vi "UHR-Fleezers Control (host) - Avogadro v3.vi"() -> ()   [LabVIEW 2014] (continued)
        n2336 = Unbundle By Name(w3621) -> ("kappa_x (pN/nm)"=w3623:dbl, "kappa_y (pN/nm)"=w3622:dbl)
        n2337 = Unbundle By Name(w3629) -> ("Set 1"=w3632:dbl, "Set 2"=w3631:dbl)
        n2338 = case shown="True" "Scale intensities" {
          tunnel: w3632 -> [w3646 w3659]
          tunnel: w3631 -> [w3645 w3652]
          tunnel: "Scaling factor" -> [w3642 w3647]
          tunnel: [w3644 w3658] -> w3627
          tunnel: [w3643 w3657] -> w3626
          tunnel: w3625 -> [w3641 w3653]
          tunnel: w3624 -> [w3640 w3654]
          tunnel: w3623 -> [w3639 w3655]
          tunnel: w3622 -> [w3638 w3656]
          tunnel: [w3637 w3651] -> w3620
          tunnel: [w3636 w3650] -> w3619
          tunnel: [w3635 w3649] -> w3618
          tunnel: [w3634 w3648] -> w3617
          frame False {
            n2339 = Divide(x=w3646, y=w3642) -> (x/y=w3644:dbl)
            n2340 = Divide(x=w3638, y=w3642) -> (x/y=w3634:dbl)
            n2341 = Divide(x=w3645, y=w3642) -> (x/y=w3643:dbl)
            n2342 = Divide(x=w3641, y=w3642) -> (x/y=w3637:dbl)
            n2343 = Divide(x=w3640, y=w3642) -> (x/y=w3636:dbl)
            n2344 = Divide(x=w3639, y=w3642) -> (x/y=w3635:dbl)
          }
          frame True {
            n2345 = Multiply(x=w3659, y=w3647) -> (x*y=w3658:dbl)
            n2346 = Multiply(x=w3652, y=w3647) -> (x*y=w3657:dbl)
            n2347 = Multiply(x=w3656, y=w3647) -> (x*y=w3648:dbl)
            n2348 = Multiply(x=w3653, y=w3647) -> (x*y=w3651:dbl)
            n2349 = Multiply(x=w3654, y=w3647) -> (x*y=w3650:dbl)
            n2350 = Multiply(x=w3655, y=w3647) -> (x*y=w3649:dbl)
          }
        }
        n2351 = Bundle By Name(cluster=w3614, "kappa_x (pN/nm)"=w3620, "kappa_y (pN/nm)"=w3619) -> (w3616:T12)
        n2352 = Bundle By Name(cluster=w3621, "kappa_x (pN/nm)"=w3618, "kappa_y (pN/nm)"=w3617) -> (w3615:T12)
        n2353 = Bundle By Name(cluster=w3629, "Set 1"=w3627, "Set 2"=w3626) -> (w3628:cluster{"Set 1":dbl, "Set 2":dbl})
        n2354 = property on="T1 calibration" class="Clust (strict)"("Val(Sgnl)"=w3616) -> ()  [unwired: 2 in, 2 out]
        n2355 = property on="T2 calibration" class="Clust (strict)"("Val(Sgnl)"=w3615) -> ()  [unwired: 2 in, 2 out]
        n2356 = property on="Setpoints (V)" class="Clust (strict)"("Val(Sgnl)"=w3628) -> ()  [unwired: 2 in, 2 out]
      }
      event "Piezo X at\n Scan position (V)": Value Change {
        n2357 = event-data() -> ()  [unwired: 7 out]
        n2358 = local read "AOM position for scan (MHz)"() -> (w3668:dbl)
        n2359 = local read "Piezo Trap X cal (nm/V)"() -> (w3662:dbl)
        n2360 = local read "AOM X Cal (nm/MHz)"() -> (w3665:dbl)
        n2361 = Subtract(x=w3668, y=60.0) -> (x-y=w3666:dbl)
        n2362 = Multiply(x=w3666, y=w3665) -> (x*y=w3663:dbl)
        n2363 = Multiply(x="Piezo X at\n Scan position (V)", y=w3662) -> (x*y=w3664:dbl)
        n2364 = Subtract(x=w3664, y=w3663) -> (x-y=w3661:dbl)
        n2365 = Divide(x=w3661, y=w3662) -> (x/y=→"Piezo trap x\noffset (V)":dbl)
      }
      event "Shift offset": Value Change {
        # "This events shifts the offset values by the currently measured values. For a quick way of correcting for changes in offsets"
        n2366 = event-data() -> ()  [unwired: 7 out]
        n2367 = local read "Multi-MCL offset array"() -> (w3691:T31)
        n2368 = local read "Offset file step size"() -> (w3679:dbl)
        n2369 = local read "MCL offset scanning range (V)"() -> (w3680:T4)
        n2370 = local write "Shift offset"(FALSE) -> ()
        n2371 = local read "Trap position array"() -> (w3692:dbl[])
        n2372 = Build Array(1, 0, 4, 3, 11, 10) -> (w3683:i32[])
        n2373 = local read "Values"() -> (w3684:dbl[])
        n2374 = for {
          tunnel: w3684 -> [w3696]
          tunnel: w3683 -> [w3695] mode=indexing
          tunnel: [w3694] -> w3682 mode=indexing
          n2375 = Index Array(array=w3696, index=w3695) -> (element=w3694:dbl)
        }
        n2376 = call "select offset array.vi"("MCL offset scanning range (V)"=w3680, "Offset File step size"=w3679, "Multi-MCL offset array"=w3691, "Trap position array"=w3692) -> ("Out offsets"=w3681:dbl[])  [unwired: 1 out]
        n2377 = Subtract(x=w3682, y=w3681) -> (x-y=w3671:dbl[])
        n2378 = local read "Raw offsets"() -> (w3678:dbl[])
        n2379 = Negate(x=w3671) -> (-x=w3670:dbl[])
        n2380 = call "generate multiple MCL offset.vi"("Offset array"=w3678, "offset file step size"=w3679, "MCL offset scanning range (V)"=w3680, "Corrections"=w3670) -> ("B_X mean out"=w3672:dbl[], "A_X mean out"=w3673:dbl[], "Output array"=w3677:T31)
        n2381 = local write "Multi-MCL offset array"(w3677) -> ()
        n2382 = local read "B factor"() -> (w3674:dbl)
        n2383 = Multiply(x=w3672, y=w3674) -> (x*y=w3676:dbl[])
        n2384 = Subtract(x=w3673, y=w3676) -> (x-y=w3675:dbl[])
        n2385 = property on="Setpoint offset\ncorrection values" class="Arr (strict)"("Val(Sgnl)"=w3675) -> ()  [unwired: 2 in, 2 out]
      }
      event "Symmetric raster\nand force FB": Value Change {
        n2386 = event-data() -> ()  [unwired: 7 out]
        n2387 = local read "Symmetric raster\nand force FB"() -> (w3697:bool)
        n2388 = xnode "Read/Write Control"("FPGA VI Reference In"=w3698, "Symmetric force feedback and raster scan"=w3697) -> ()  [unwired: 1 in, 2 out]
      }
      event "EMCCD Gate", "EMCCD Gate ON Count", "EMCCD Gate OFF Count", "Invert EMCCD Gate": Value Change {
        n2389 = event-data() -> ()  [unwired: 7 out]
        n2390 = xnode "Read/Write Control"("FPGA VI Reference In"=w3703, "EMCCD Gate ON count"="EMCCD Gate ON Count", "EMCCD Gate OFF count"="EMCCD Gate OFF Count", "Invert EMCCD Gate"="Invert EMCCD Gate", "EMCCD Gate Operating Mode"="EMCCD Gate") -> ()  [unwired: 1 in, 2 out]
      }
      event "+ phase (EMCCD Gate)", "- phase (EMCCD Gate)": Value Change {
        n2391 = event-data() -> ()  [unwired: 7 out]
        n2392 = Or(x="- phase (EMCCD Gate)", y="+ phase (EMCCD Gate)") -> (x .or. y?=w3708:bool)
        n2393 = Negate(x="Phase Adj. (EMCCD Gate)") -> (-x=w3714:i16)
        n2394 = Select(t=w3714, s="+ phase (EMCCD Gate)", f="Phase Adj. (EMCCD Gate)") -> (s? t:f=w3709:i16)
        n2395 = flat-sequence {
          tunnel: w3710 -> [w3718]
          tunnel: w3709 -> [w3717]
          tunnel: [w3716] -> w3707
          tunnel: [w3715] -> w3705
          tunnel: w3708 -> [w3715]
          tunnel: w3707 -> [w3721]
          tunnel: [w3721] -> w3706
          tunnel: w3705 -> [w3720]
          tunnel: [w3720] -> w3704
          tunnel: w3706 -> [w3723]
          tunnel: w3704 -> [w3722]
          frame #0 {
            n2396 = xnode "Read/Write Control"("FPGA VI Reference In"=w3718, "Phase Count Adjustment EMCCD Gate"=w3717) -> ("FPGA VI Reference Out"=w3716:T41)  [unwired: 1 in, 1 out]
          }
          frame #1 {
            n2397 = Wait (ms)(milliseconds to wait=100) -> ()  [unwired: 1 out]
          }
          frame #2 {
            n2398 = xnode "Read/Write Control"("FPGA VI Reference In"=w3723, "+ phase (EMCCD Gate)"=w3722) -> ()  [unwired: 1 in, 2 out]
          }
        }
      }
    }
    "error out 2" <- w1836
    n2399 = node-c288() -> ()  [unwired: 2 out]
  }
  n2400 = node-c288() -> (w64:T43)  [unwired: 4 out]
  n2401 = timed-loop "Mouse control: trap position (AOM deflection), set confocal spot from image" {
    tunnel: [w3724] -> w69
    timing: w64 -> [_]
    timing-out: [_] -> w63
    tunnel: w26 -> [w3725]
    stop <- w3724 stop-if-true
    n2402 = node-c288() -> ()  [unwired: 2 out]
    n2403 = event shown="[0] \"Pane\": Mouse Down" {
      selector: _ -> [_ _ _ _]
      dyn-events: _ -> [_ _ _ _]
      timeout: _ -> [_ _ _ _]
      tunnel: w3725 -> [w3728 _ _ _]
      tunnel: [_ _ TRUE _] -> w3724
      event Mouse Down {
        n2404 = event-data() -> ("Time"=w3730:u32, "Coords"=w3729:T16, "Button"=w3731:u16)  [unwired: 6 out]
        n2405 = case shown="1" w3731 {
          tunnel: w3730 -> [_ _ w3861]
          tunnel: w3729 -> [_ w3768 w3859]
          tunnel: w3728 -> [_ _ w3855]
          frame 0, Default {
          }
          frame 1 {
            n2406 = property on="APD 2" class="ImageControl"() -> ("Displayed Image Position"=w3738:cluster{"Left":i32, "Top":i32})  [unwired: 2 in, 2 out]
            n2407 = property on="APD 1" class="ImageControl"() -> ("Displayed Image Position"=w3767:cluster{"Left":i32, "Top":i32})  [unwired: 2 in, 2 out]
            n2408 = property on="Detection Laser X" class="ImageControl"() -> ("Displayed Image Position"=w3764:cluster{"Left":i32, "Top":i32})  [unwired: 2 in, 2 out]
            n2409 = property on="Detection Laser Y" class="ImageControl"() -> ("Displayed Image Position"=w3763:cluster{"Left":i32, "Top":i32})  [unwired: 2 in, 2 out]
            n2410 = property on="APD 2" class="ImageControl"() -> ("Displayed Image Size"=w3737:cluster{"Width":u32, "Height":u32})  [unwired: 2 in, 2 out]
            n2411 = property on="APD 1" class="ImageControl"() -> ("Displayed Image Size"=w3765:cluster{"Width":u32, "Height":u32})  [unwired: 2 in, 2 out]
            n2412 = property on="Detection Laser X" class="ImageControl"() -> ("Displayed Image Size"=w3766:cluster{"Width":u32, "Height":u32})  [unwired: 2 in, 2 out]
            n2413 = property on="Detection Laser Y" class="ImageControl"() -> ("Displayed Image Size"=w3762:cluster{"Width":u32, "Height":u32})  [unwired: 2 in, 2 out]
            n2414 = Unbundle By Name(w3737) -> ("Width"=w3734:u32, "Height"=w3733:u32)
            n2415 = Unbundle By Name(w3738) -> ("Left"=w3736:i32, "Top"=w3735:i32)
            n2416 = Unbundle By Name(w3765) -> ("Width"=w3759:u32, "Height"=w3758:u32)
            n2417 = Unbundle By Name(w3766) -> ("Width"=w3755:u32, "Height"=w3754:u32)
            n2418 = Unbundle By Name(w3762) -> ("Width"=w3751:u32, "Height"=w3750:u32)
            n2419 = Unbundle By Name(w3767) -> ("Left"=w3761:i32, "Top"=w3760:i32)
            n2420 = Unbundle By Name(w3764) -> ("Left"=w3757:i32, "Top"=w3756:i32)
            n2421 = Unbundle By Name(w3763) -> ("Left"=w3753:i32, "Top"=w3752:i32)
            n2422 = Bundle("Left"=w3736, "Top"=w3735, "Width"=w3734, "Height"=w3733) -> (w3732:T59)  [unwired: 1 in]
            n2423 = Bundle("Left"=w3761, "Top"=w3760, "Width"=w3759, "Height"=w3758) -> (w3749:T59)  [unwired: 1 in]
            n2424 = Bundle("Left"=w3757, "Top"=w3756, "Width"=w3755, "Height"=w3754) -> (w3748:T59)  [unwired: 1 in]
            n2425 = Bundle("Left"=w3753, "Top"=w3752, "Width"=w3751, "Height"=w3750) -> (w3747:T59)  [unwired: 1 in]
            n2426 = Build Cluster Array(w3732, w3749, w3748, w3747) -> (w3746:T60)
            n2427 = for {
              tunnel: w3768 -> [w3779]
              tunnel: w3746 -> [w3780] mode=indexing
              shift-right: [w3777] -> w3744
              shift-left: TRUE -> [w3778]
              shift-right: [w3776] -> w3742
              shift-left: _ -> [w3772]
              shift-right: [w3775] -> w3741
              shift-left: _ -> [w3771]
              shift-right: [w3774] -> w3740
              shift-left: _ -> [w3770]
              shift-right: [w3773] -> w3739
              shift-left: _ -> [w3769]
              n2428 = case shown="True" w3778 {
                selector: w3778 -> [w3785 _]
                tunnel: w3780 -> [_ w3794]
                tunnel: w3779 -> [_ w3792]
                tunnel: [w3785 w3790] -> w3777
                tunnel: [w3784 w3789] -> w3776
                tunnel: [w3783 w3788] -> w3775
                tunnel: [w3782 w3787] -> w3774
                tunnel: [w3781 w3786] -> w3773
                tunnel: w3772 -> [w3784 _]
                tunnel: w3771 -> [w3783 _]
                tunnel: w3770 -> [w3782 _]
                tunnel: w3769 -> [w3781 _]
                frame False {
                }
                frame True {
                  n2429 = Unbundle(w3794) -> (w3793:T59)
                  n2430 = call "isclickinwindow.vi"("Image Param"=w3793, "Point32"=w3792) -> ("4 Y"=w3786:i32, "3 Height"=w3787:i32, "2 X"=w3788:i32, "1 Width"=w3789:i32, "In image?"=w3791:bool)  [unwired: 1 in]
                  n2431 = Not(x=w3791) -> (.not. x?=w3790:bool)
                }
              }
            }
            n2432 = Not(x=w3744) -> (.not. x?=w3743:bool)
            n2433 = case shown="True" w3743 {
              tunnel: w3741 -> [_ w3820]
              tunnel: w3739 -> [_ w3819]
              tunnel: w3742 -> [_ w3818]
              tunnel: w3740 -> [_ w3817]
              frame False {
              }
              frame True {
                w3807 = FALSE ("Get Point")
                n2434 = local read "Scan lines (y)"() -> (w3800:u64)
                n2435 = local read "Initial Y"() -> (w3798:dbl)
                n2436 = local read "Actual MCL Inc (V)"() -> (w3801:dbl)
                n2437 = local read "Scan steps (MCL)"() -> (w3804:u64)
                n2438 = local read "Actual MCL Inc (V)"() -> (w3816:dbl)
                n2439 = local read "Scan lines (y)"() -> (w3821:u64)
                n2440 = Divide "Y Pix/step"(x=w3817, y=w3821) -> (x/y=w3827:dbl)
                n2441 = Multiply(x=w3801, y=w3800) -> (x*y=w3799:dbl)
                n2442 = Divide "X pix/step"(x=w3818, y=w3804) -> (x/y=w3825:dbl)
                n2443 = Add(x=w3799, y=w3798) -> (x+y=w3797:dbl)
                n2444 = Divide "Y V/pix"(x=w3816, y=w3827) -> (x/y=w3826:dbl)
                n2445 = Divide "Y half step offset"(x=w3816, y=2.0) -> (x/y=w3803:dbl)
                n2446 = Divide "X half step offset"(x=w3816, y=2.0) -> (x/y=w3823:dbl)
                n2447 = Divide "X V/pix"(x=w3816, y=w3825) -> (x/y=w3824:dbl)
                n2448 = Multiply(x=w3819, y=w3826) -> (x*y=w3796:dbl)
                n2449 = Negate(x=w3796) -> (-x=w3795:dbl)
                n2450 = Negate(x=w3803) -> (-x=w3802:dbl)
                n2451 = Multiply(x=w3816, y=w3804) -> (x*y=w3829:dbl)
                n2452 = Multiply(x=w3824, y=w3820) -> (x*y=w3831:dbl)
                n2453 = Negate(x=w3823) -> (-x=w3822:dbl)
                n2454 = Compound Arithmetic op=ADD(w3802, w3795, w3797) -> (w3808:dbl)
                "Pointer Y (V)" <- w3808
                n2455 = local read "Initial X"() -> (w3832:dbl)
                n2456 = Negate(x=w3831) -> (-x=w3830:dbl)
                n2457 = Compound Arithmetic op=ADD(w3822, w3829, w3832, w3830) -> (w3809:dbl)
                "Pointer X (V)" <- w3809
                n2458 = case shown="True" "Set High F Confocal Spot (X-Y)" {
                  tunnel: w3809 -> [_ w3853]
                  tunnel: w3808 -> [_ w3854]
                  frame False {
                  }
                  frame True {
                    "Confocal Y 2 (V)" <- w3854
                    "Confocal X 2 (V)" <- w3853
                  }
                }
                n2459 = local read "Scan trap 3 or Fl?"() -> (w3806:bool)
                n2460 = Or(x="Set X Only", y="Set Confocal Spot (X-Y)") -> (x .or. y?=w3812:bool)
                n2461 = Or(x="Set Confocal Spot (X-Y)", y="Set Y Only") -> (x .or. y?=w3811:bool)
                n2462 = case shown="False" w3806 {
                  tunnel: w3812 -> [w3836 w3842]
                  tunnel: w3811 -> [w3835 w3841]
                  tunnel: w3809 -> [w3834 w3839]
                  tunnel: w3808 -> [w3833 w3840]
                  frame False {
                    n2463 = case shown="True" w3835 {
                      tunnel: w3833 -> [_ w3838]
                      frame False {
                      }
                      frame True {
                        n2464 = property on="AO1" class="Slide (strict)"("Val(Sgnl)"=w3838) -> ()  [unwired: 2 in, 2 out]
                        "Confocal Y 1 (V)" <- w3838
                      }
                    }
                    n2465 = case shown="True" w3836 {
                      tunnel: w3834 -> [_ w3837]
                      frame False {
                      }
                      frame True {
                        n2466 = property on="AO2" class="Slide (strict)"("Val(Sgnl)"=w3837) -> ()  [unwired: 2 in, 2 out]
                        "Confocal X 1 (V)" <- w3837
                      }
                    }
                  }
                  frame True {
                    n2467 = case shown="True" w3841 {
                      tunnel: w3840 -> [_ w3843]
                      frame False {
                      }
                      frame True {
                        n2468 = property on="Piezo trap y\noffset (V)" class="DigNum (strict)"("Val(Sgnl)"=w3843) -> ()  [unwired: 2 in, 2 out]
                      }
                    }
                    n2469 = case shown="True" w3842 {
                      tunnel: w3839 -> [_ w3848]
                      frame False {
                      }
                      frame True {
                        n2470 = local read "AOM X Cal (nm/MHz)"() -> (w3849:dbl)
                        n2471 = local read "Trap Delta (MHz)"() -> (w3851:dbl)
                        n2472 = Subtract(x=30.0, y=w3851) -> (x-y=w3850:dbl)
                        n2473 = Multiply(x=w3850, y=w3849) -> (x*y=w3846:dbl)
                        n2474 = local read "Piezo Trap X cal (nm/V)"() -> (w3845:dbl)
                        n2475 = Divide(x=w3846, y=w3845) -> (x/y=w3844:dbl)
                        n2476 = Subtract(x=w3848, y=w3844) -> (x-y=w3847:dbl)
                        n2477 = property on="Piezo trap x\noffset (V)" class="DigNum (strict)"("Val(Sgnl)"=w3847) -> ()  [unwired: 2 in, 2 out]
                      }
                    }
                  }
                }
                n2478 = local write "Set High F Confocal Spot (X-Y)"(w3807) -> ()
                n2479 = local write "Set Confocal Spot (X-Y)"(w3807) -> ()
                n2480 = local write "Set X Only"(w3807) -> ()
                n2481 = local write "Set Y Only"(w3807) -> ()
              }
            }
          }
          frame 3 {
            n2482 = local read "BD 2 Frequency 1 (MHz)"() -> (w3856:dbl)
            n2483 = local read "BD 1 Frequency 1 (MHz)"() -> (w3857:dbl)
            n2484 = local write "Manipulating Trap"(TRUE ("Manipulating Trap")) -> ()
            n2485 = local write "Coords"(T16 {"Horizontal"=0, "Vertical"=0} ("Coords")) -> ()
            n2486 = while {
              tunnel: w3861 -> [w3866]
              tunnel: w3859 -> [w3865]
              tunnel: w3857 -> [w3864]
              tunnel: w3856 -> [w3863]
              tunnel: w3855 -> [w3862]
              stop <- w3867 stop-if-true
              n2487 = event shown="[0] \"Pane\": Mouse Move" {
                selector: _ -> [_ _]
                dyn-events: _ -> [_ _]
                timeout: _ -> [_ _]
                tunnel: ["Force Manip Abort" w3931] -> w3867
                tunnel: w3866 -> [w3874 _]
                tunnel: w3865 -> [w3872 _]
                tunnel: w3864 -> [w3871 _]
                tunnel: w3863 -> [w3870 _]
                tunnel: w3862 -> [w3868 _]
                event Mouse Move {
                  n2488 = event-data() -> ("Time"=w3875:u32, "Coords"=w3876:T16)  [unwired: 3 out]
                  n2489 = Less?(x=w3875, y=w3874) -> (x < y?=w3873:bool)
                  n2490 = case "Makes sure old motion events prior to mouse click aren't used" shown="False" w3873 {
                    tunnel: w3876 -> [w3918 _]
                    tunnel: w3872 -> [w3919 _]
                    tunnel: w3871 -> [w3893 _]
                    tunnel: w3870 -> [w3892 _]
                    tunnel: w3868 -> [w3877 _]
                    frame False {
                      n2491 = Subtract(x=w3918, y=w3919) -> (x-y=w3917:T16)
                      "Coords" <- w3917
                      n2492 = local read "Y RF Frequency Limits (MHz)"() -> (w3878:T27)
                      n2493 = To Double Precision Float(number=w3917) -> (double precision float=w3916:cluster{"Horizontal":dbl, "Vertical":dbl})
                      n2494 = Multiply(x=cluster{"Horizontal":dbl, "Vertical":dbl} {"Horizontal"=-1.0, "Vertical"=1.0}, y="Manipulation Scaling") -> (x*y=w3912:cluster{"Horizontal":dbl, "Vertical":dbl})
                      n2495 = local read "X RF Frequency Limits (MHz)"() -> (w3879:T27)
                      n2496 = Multiply(x=w3916, y=w3912) -> (x*y=w3914:cluster{"Horizontal":dbl, "Vertical":dbl})
                      n2497 = Unbundle By Name(w3914) -> ("Horizontal"=w3909:dbl, "Vertical"=w3913:dbl)
                      n2498 = Unbundle By Name(w3878) -> ("Maximum"=w3881:dbl, "Minimum"=w3880:dbl)
                      n2499 = Boolean To (0,1)(Boolean="Manip. X?") -> (0, 1=w3907:i16)
                      n2500 = Boolean To (0,1)(Boolean="Manip. Y?") -> (0, 1=w3904:i16)
                      n2501 = local read "BD 1 Frequency 2 (MHz)"() -> (w3895:dbl)
                      n2502 = Multiply(x=w3913, y=w3904) -> (x*y=w3906:dbl)
                      n2503 = Multiply(x=w3907, y=w3909) -> (x*y=w3910:dbl)
                      n2504 = local read "BD 2 Frequency 2 (MHz)"() -> (w3894:dbl)
                      n2505 = Unbundle By Name(w3879) -> ("Maximum"=w3883:dbl, "Minimum"=w3882:dbl)
                      n2506 = Add(x=w3892, y=w3906) -> (x+y=w3885:dbl)
                      n2507 = Add(x=w3893, y=w3910) -> (x+y=w3887:dbl)
                      n2508 = In Range and Coerce(upper limit=w3883, x=w3887, lower limit=w3882) -> (coerced(x)=w3886:dbl)  [unwired: 1 out]
                      n2509 = In Range and Coerce(upper limit=w3881, x=w3885, lower limit=w3880) -> (coerced(x)=w3884:dbl)  [unwired: 1 out]
                      n2510 = Subtract(x=w3886, y=w3895) -> (x-y=w3903:dbl)
                      n2511 = Subtract(x=w3884, y=w3894) -> (x-y=w3902:dbl)
                      n2512 = Square(x=w3903) -> (x^2=w3901:dbl)
                      n2513 = Square(x=w3902) -> (x^2=w3900:dbl)
                      n2514 = Add(x=w3901, y=w3900) -> (x+y=w3899:dbl)
                      n2515 = Square Root(x=w3899) -> (sqrt(x)=w3896:dbl)
                      n2516 = In Range and Coerce(upper limit="Limit Max (MHz)", x=w3896, lower limit="Limit Min (MHz)") -> (In Range?=w3889:bool)  [unwired: 1 out]
                      n2517 = Not(x="Limits Enable") -> (.not. x?=w3888:bool)
                      n2518 = Or(x=w3889, y=w3888) -> (x .or. y?=w3890:bool)
                      n2519 = case shown="True" w3890 {
                        tunnel: w3896 -> [_ w3921]
                        tunnel: w3886 -> [_ w3928]
                        tunnel: w3895 -> [_ w3927]
                        tunnel: w3884 -> [_ w3926]
                        tunnel: w3894 -> [_ w3925]
                        tunnel: w3879 -> [_ w3923]
                        tunnel: w3878 -> [_ w3922]
                        tunnel: w3877 -> [_ w3920]
                        frame False {
                        }
                        frame True {
                          n2520 = local read "BD 1 Frequency 3 (MHz)"() -> (w3929:dbl)
                          n2521 = local read "BD 2 Frequency 3 (MHz)"() -> (w3924:dbl)
                          n2522 = local write "Trap Delta (MHz)"(w3921) -> ()
                          n2523 = call "set RF board frequency - interlace.vi"("Board 2 Frequency Limits"=w3922, "Board 1 Frequency Limits"=w3923, "FPGA VI Reference In"=w3920, "Board 2 Frequency 3 (MHz)"=w3924, "Board 1 Frequency 3 (MHz)"=w3929, "Board 2 Frequency 2 (MHz)"=w3925, "Board 2 Frequency 1 (MHz)"=w3926, "Board 1 Frequency 2 (MHz)"=w3927, "Board 1 Frequency 1  (MHz)"=w3928) -> ()  [unwired: 1 in, 2 out]
                          n2524 = local write "BD 2 Frequency 1 (MHz)"(w3926) -> ()
                          n2525 = local write "BD 1 Frequency 1 (MHz)"(w3928) -> ()
                        }
                      }
                    }
                    frame True {
                    }
                  }
                }
                event Mouse Up {
                  n2526 = event-data() -> ("Button"=w3930:u16)  [unwired: 8 out]
                  n2527 = case shown="3" w3930 {
                    tunnel: [FALSE TRUE] -> w3931
                    frame 0, Default {
                    }
                    frame 3 {
                      n2528 = local read "Trap Delta (MHz)"() -> (w3933:dbl)
                      n2529 = property on="Initial delta (MHz)" class="DigNum (strict)"("Val(Sgnl)"=w3933) -> ()  [unwired: 2 in, 2 out]
                      n2530 = local write "Manipulating Trap"(FALSE ("Manipulating Trap")) -> ()
                    }
                  }
                }
              }
            }
          }
        }
      }
      event Timeout {
        n2531 = event-data() -> ()  [unwired: 4 out]
      }
      event "Stop All": Mouse Down {
        n2532 = event-data() -> ()  [unwired: 9 out]
      }
      event Mouse Move {
        n2533 = event-data() -> ()  [unwired: 6 out]
      }
    }
    n2534 = node-c288() -> ()  [unwired: 2 out]
  }
  n2535 = node-c288(i64 1 ("Period"), 1 ("Processor")) -> (w68:T43)  [unwired: 2 in, 2 out]
  n2536 = node-c288(3 ("Processor")) -> (w60:T43)  [unwired: 3 out]
  n2537 = timed-loop "Oscillate Trap/AOM (fishing, conjugate plane alignment)" {
    tunnel: [w3939] -> w65
    timing: w60 -> [_]
    timing-out: [_] -> w59
    tunnel: w26 -> [w3938]
    tunnel: w3 -> [w3937]
    stop <- w3939 stop-if-true
    n2538 = node-c288() -> ()  [unwired: 2 out]
    n2539 = event shown="[2] \"Start assembly line\": Value Change" {
      selector: _ -> [_ _ _ _]
      dyn-events: _ -> [_ _ _ _]
      timeout: _ -> [_ _ _ _]
      tunnel: [FALSE ("Stop All") _ _ w4612] -> w3939
      tunnel: w3938 -> [w3942 _ _ _]
      tunnel: w3937 -> [_ _ w4547 _]
      event "Oscillate Set 1", "Fish for Tether": Value Change {
        n2540 = event-data() -> ()  [unwired: 6 out]
        n2541 = local read "Oscillate Set 1"() -> (w3946:bool)
        n2542 = Or(x=w3946, y="Fish for Tether") -> (x .or. y?=w3944:bool)
        n2543 = case shown="True" w3944 {
          tunnel: "Fish for Tether" -> [_ w3949]
          tunnel: w3942 -> [_ w3947]
          frame False {
          }
          frame True {
            n2544 = case shown="True" w3949 {
              selector: w3949 -> [w3952 w3958]
              tunnel: [w3952 w3958] -> w3948
              frame False {
              }
              frame True {
                n2545 = local write "Scan axis 2"(TRUE) -> ()
                n2546 = local write "Tether"(FALSE ("Tether")) -> ()
                n2547 = local read "Flow ON during cal?"() -> (w3953:bool)
                n2548 = property on="Trap Delta (MHz)" class="DigNum (strict)"("Val(Sgnl)"="Furthest Delta (MHz)") -> ()  [unwired: 2 in, 2 out]
                n2549 = Or(x="Flow ON during \nfishing?", y=w3953) -> (x .or. y?=w3954:bool)
                n2550 = Wait (ms)(milliseconds to wait=u32 500) -> ()  [unwired: 1 out]
                n2551 = property on="Sample Channel\nFlow" class="Bool (strict)"("Val(Sgnl)"=w3954) -> ()  [unwired: 2 in, 2 out]
              }
            }
            n2552 = node-c288() -> (w3951:T43)  [unwired: 1 in, 3 out]
            n2553 = timed-loop "Oscillate AOD" {
              timing: w3951 -> [_]
              timing-out: [_] -> w3950
              tunnel: w3948 -> [w3962]
              tunnel: w3947 -> [w3961]
              i -> [w3970]
              stop <- w3968 stop-if-true
              n2554 = node-c288() -> (w3969:i64)  [unwired: 1 out]
              n2555 = flat-sequence {
                tunnel: w3970 -> [w3997]
                tunnel: w3969 -> [w3996]
                tunnel: w3962 -> [w3980]
                tunnel: [w3980] -> w3967
                tunnel: [w3979] -> w3966
                tunnel: [w3978] -> w3965
                tunnel: [w3975] -> w3963
                tunnel: w3961 -> [w3971]
                tunnel: w3967 -> [w4044]
                tunnel: w3966 -> [w4042]
                tunnel: w3965 -> [w4041]
                tunnel: [w4040] -> w3964
                tunnel: w3963 -> [w4039]
                tunnel: [w4116] -> w3968
                tunnel: w3964 -> [w4115]
                frame #0 {
                  # "w (rad/s)"
                  # "t (s)"
                  n2556 = Divide(x=w3996, y=i64 1000) -> (x/y=w3972:dbl)
                  n2557 = local read "BD 1 Frequency 2 (MHz)"() -> (w3974:dbl)
                  n2558 = Multiply(x="Osc. freq. (Hz)", y=6.283185307179586) -> (x*y=w3994:dbl)
                  n2559 = Multiply(x=w3972, y=w3997) -> (x*y=w3993:dbl)
                  n2560 = Multiply(x=w3994, y=w3993) -> (x*y=w3977:dbl)
                  n2561 = local read "BD 1 Frequency 1 (MHz)"() -> (w3982:dbl)
                  n2562 = case shown="True" w3980 {
                    tunnel: w3977 -> [w4003 w4022]
                    tunnel: w3982 -> [_ w4030]
                    tunnel: w3974 -> [_ w4031]
                    tunnel: [w4000 w4026] -> w3973
                    tunnel: [FALSE w4004] -> w3978
                    tunnel: [0.0 w4018] -> w3975
                    frame False {
                      n2563 = Sine(x=w4003) -> (sin(x)=w4001:dbl)
                      n2564 = Multiply(x=w4001, y="Osc. amp. (MHz)") -> (x*y=w4000:dbl)
                    }
                    frame True {
                      # "trap position goes from 0 to 1 (0 is when it is furthest away, 1 is when closest)\nso we want to test for tether only when farther away, or x < 1"
                      # "quit if taking too long"
                      # "oscillate the trap"
                      # "Test for tether"
                      n2565 = local read "Vec Mean of T1 T2"() -> (w4007:dbl[])
                      "Trigger Signal" <- w4007
                      n2566 = Cosine(x=w4022) -> (cos(x)=w4034:dbl)
                      n2567 = Subtract(x=w4031, y=w4030) -> (x-y=w4029:dbl)
                      n2568 = Decrement(x=w4034) -> (x-1=w4033:dbl)
                      n2569 = Subtract(x=w4029, y="Closest Delta (MHz)") -> (x-y=w4027:dbl)
                      n2570 = Divide(x=w4033, y=-2.0) -> (x/y=w4017:dbl)
                      n2571 = Greater?(x=w4007, y="Stop F (pN)") -> (0:w4024:bool[])
                      n2572 = Multiply(x=w4017, y=w4027) -> (x*y=w4026:dbl)
                      n2573 = Less?(x=w4017, y="Fish mask thresh") -> (x < y?=w4016:bool)
                      n2574 = Boolean To (0,1)(Boolean=w4016) -> (0, 1=w4014:i16)
                      n2575 = Multiply(x=w4014, y=w4007) -> (x*y=w4013:dbl[])
                      n2576 = Divide(x=w4022, y=6.283185307179586) -> (x/y=w4021:dbl)
                      n2577 = Round Toward +Infinity(x=w4021) -> (ceil(x): smallest int >= x=w4018:dbl)
                      "Attempts" <- w4018
                      n2578 = Greater?(x=w4013, y="Stop F (pN) (mask)") -> (0:w4011:bool[])
                      n2579 = Or Array Elements(Boolean array=w4024) -> (logical OR=w4009:bool)
                      n2580 = Or Array Elements(Boolean array=w4011) -> (logical OR=w4008:bool)
                      n2581 = Greater?(x=w4018, y="Attempt Limit") -> (0:w4020:bool)
                      n2582 = case shown="True" w4020 {
                        frame False {
                        }
                        frame True {
                          n2583 = local write "Fish for Tether"(FALSE ("Fish for Tether")) -> ()
                          n2584 = call <vilib>:"Beep.vi"() -> ()  [unwired: 3 in, 9 out]
                          n2585 = local read "Messages"() -> (w4036:string)
                          n2586 = call "Update messages.vi"("Message to add"="Tether fishing timeout." ("Messages"), "Old message string"=w4036) -> ("New message string"=→"Messages":string)
                        }
                      }
                      n2587 = Select(t=w4009, s="Normal (on) or masked test (off)", f=w4008) -> (s? t:f=w4006:bool)
                      n2588 = And(x="Stop Fishing When Tether", y=w4006) -> (x .and. y?=w4004:bool)
                    }
                  }
                  n2589 = local read "BD 2 Frequency 1 (MHz)"() -> (w3981:dbl)
                  n2590 = Select(t=w3982, s="Scan axis 2", f=w3981) -> (s? t:f=w3985:dbl)
                  n2591 = Add(x=w3973, y=w3985) -> (x+y=w3979:dbl)
                  n2592 = Select(t=w3979, s="Scan axis 2", f=w3982) -> (s? t:f=w3988:dbl)
                  n2593 = Select(t=w3981, s="Scan axis 2", f=w3979) -> (s? t:f=w3987:dbl)
                  n2594 = local read "BD 2 Frequency 2 (MHz)"() -> (w3990:dbl)
                  n2595 = local read "BD 2 Frequency 3 (MHz)"() -> (w3989:dbl)
                  n2596 = local read "Y RF Frequency Limits (MHz)"() -> (w3983:T27)
                  n2597 = local read "X RF Frequency Limits (MHz)"() -> (w3984:T27)
                  n2598 = local read "BD 1 Frequency 3 (MHz)"() -> (w3991:dbl)
                  n2599 = call "set RF board frequency - interlace.vi"("Board 2 Frequency Limits"=w3983, "Board 1 Frequency Limits"=w3984, "FPGA VI Reference In"=w3971, "Board 2 Frequency 3 (MHz)"=w3989, "Board 1 Frequency 3 (MHz)"=w3991, "Board 2 Frequency 2 (MHz)"=w3990, "Board 2 Frequency 1 (MHz)"=w3987, "Board 1 Frequency 2 (MHz)"=w3974, "Board 1 Frequency 1  (MHz)"=w3988) -> ()  [unwired: 1 in, 2 out]
                }
                frame #1 {
                  n2600 = And(x=w4044, y=w4041) -> (x .and. y?=w4043:bool)
                  n2601 = case "Only if were fishing and now formed tether" shown="True" w4043 {
                    tunnel: w4042 -> [w4046 w4061]
                    tunnel: [w4045 w4060] -> w4040
                    tunnel: w4039 -> [_ w4056]
                    frame False {
                      n2602 = local read "Fish for Tether"() -> (w4045:bool)
                      n2603 = case shown="False" w4045 {
                        tunnel: w4046 -> [w4047 _]
                        frame False {
                          n2604 = property on="BD 1 Frequency 1 (MHz)" class="DigNum (strict)"("Val(Sgnl)"=w4047) -> ()  [unwired: 2 in, 2 out]
                        }
                        frame True {
                        }
                      }
                    }
                    frame True {
                      w4060 = FALSE ("Fish for Tether")
                      n2605 = call <vilib>:"Beep.vi"() -> ()  [unwired: 3 in, 9 out]
                      n2606 = Number To Decimal String(number=w4056, width (-)=i16 1) -> (decimal integer string=w4054:string)
                      n2607 = Concatenate Strings("Formed tether in ", w4054, " attempt(s)." ("string")) -> (w4051:string)
                      n2608 = local read "Messages"() -> (w4058:string)
                      n2609 = local write "Fish for Tether"(w4060) -> ()
                      n2610 = call "Update messages.vi"("Message to add"=w4051, "Old message string"=w4058) -> ("New message string"=w4057:string)
                      n2611 = local write "Messages"(w4057) -> ()
                      n2612 = Get Date/Time In Seconds() -> (seconds since 1Jan1904=→"Time tether formed":timestamp)
                      n2613 = local read "Flow ON during cal?"() -> (w4048:bool)
                      n2614 = property on="Sample Channel\nFlow" class="Bool (strict)"("Val(Sgnl)"=w4048) -> (error out=w4049:errorcluster)  [unwired: 2 in, 1 out]
                      n2615 = case shown="\"2\", \"3\", \"4\", \"5\", \"6\"" "Then..." {
                        selector: "Then..." -> [_ w4064]
                        tunnel: w4061 -> [w4063 _]
                        tunnel: w4049 -> [_ _]
                        frame "1", Default {
                          n2616 = property on="BD 1 Frequency 1 (MHz)" class="DigNum (strict)"("Val(Sgnl)"=w4063) -> ()  [unwired: 2 in, 2 out]
                        }
                        frame "2", "3", "4", "5", "6" {
                          n2617 = flat-sequence {
                            tunnel: w4064 -> [w4066]
                            frame #0 {
                              n2618 = property on="Trap Delta (MHz)" class="DigNum (strict)"("Val(Sgnl)"="Move to Delta 1 (MHz)") -> ()  [unwired: 2 in, 2 out]
                            }
                            frame #1 {
                              n2619 = case shown="\"5\", \"6\"" w4066 {
                                selector: w4066 -> [w4069 w4079 _]
                                frame "3", "4" {
                                n2620 = flat-sequence {
                                tunnel: w4069 -> [w4070]
                                tunnel: [w4070] -> w4067
                                tunnel: [w4072] -> w4068
                                tunnel: w4067 -> [w4072]
                                tunnel: w4068 -> [w4076]
                                frame #0 {
                                n2621 = property on="Vortran Laser ON" class="Bool (strict)"("Val(Sgnl)"=TRUE ("Value (Signaling)")) -> ()  [unwired: 2 in, 2 out]
                                }
                                frame #1 {
                                n2622 = Multiply(x="Wait Before Save (s)", y=u32 1000 ("x")) -> (x*y=w4074:u32)
                                n2623 = Wait (ms)(milliseconds to wait=w4074) -> ()  [unwired: 1 out]
                                }
                                frame #2 {
                                n2624 = property on="Start Saving" class="Bool (strict)"("Value"=TRUE ("Start Saving")) -> ()  [unwired: 2 in, 2 out]
                                n2625 = case shown="\"4\"" w4076 {
                                frame Default {
                                }
                                frame "4" {
                                n2626 = property on="Fl. Triggered..." class="Bool (strict)"("Val(Sgnl)"=TRUE ("Value (Signaling)")) -> ()  [unwired: 2 in, 2 out]
                                }
                                }
                                }
                                }
                                }
                                frame "5", "6" {
                                n2627 = stacked-sequence {
                                tunnel: w4079 -> [_ _ _ _ _ _ w4091]
                                frame #0 {
                                n2628 = Replace Array Subset(array=u32[] [0] ("Index Values"), new element="Raster Set Upon Tether", index=0) -> (w4080:u32[])
                                n2629 = property on="Saved AOD Raster Scan Parameter Sets" class="Arr (strict)"("Index Values"=w4080) -> ()  [unwired: 2 in, 2 out]
                                }
                                frame #1 {
                                n2630 = Wait (ms)(milliseconds to wait=u32 500) -> ()  [unwired: 1 out]
                                }
                                frame #2 {
                                n2631 = property on="Load parameters" class="Bool (strict)"("Val(Sgnl)"=TRUE ("Value (Signaling)")) -> ()  [unwired: 2 in, 2 out]
                                n2632 = case shown="True" "Green ON During Raster" {
                                frame False {
                                }
                                frame True {
                                n2633 = property on="Vortran Laser ON" class="Bool (strict)"("Val(Sgnl)"=TRUE ("Value (Signaling)")) -> ()  [unwired: 2 in, 2 out]
                                }
                                }
                                }
                                frame #3 {
                                n2634 = Wait (ms)(milliseconds to wait=u32 500) -> ()  [unwired: 1 out]
                                }
                                frame #4 {
                                n2635 = property on="Trap Raster Scan" class="Bool (strict)"("Val(Sgnl)"=TRUE ("Value (Signaling)")) -> ()  [unwired: 2 in, 2 out]
                                }
                                frame #5 {
                                n2636 = Wait (ms)(milliseconds to wait=u32 2000) -> ()  [unwired: 1 out]
                                }
                                frame #6 {
                                n2637 = flat-sequence {
                                tunnel: w4091 -> [w4098]
                                frame #0 {
                                n2638 = while {
                                stop <- w4094 stop-if-true
                                n2639 = local read "Raster Scanning..."() -> (w4093:bool)
                                n2640 = local read "Saving..."() -> (w4096:bool)
                                n2641 = Wait (ms)(milliseconds to wait=u32 100) -> ()  [unwired: 1 out]
                                n2642 = Not(x=w4096) -> (.not. x?=w4095:bool)
                                n2643 = Not(x=w4093) -> (.not. x?=w4092:bool)
                                n2644 = And(x=w4095, y=w4092) -> (x .and. y?=w4094:bool)
                                }
                                }
                                frame #1 {
                                n2645 = local read "Tether"() -> (w4099:bool)
                                n2646 = case shown="True" w4099 {
                                tunnel: w4098 -> [_ w4101]
                                frame False {
                                n2647 = property on="Fish for Tether" class="Bool (strict)"("Val(Sgnl)"="Fish again after \nraster break?") -> ()  [unwired: 2 in, 2 out]
                                }
                                frame True {
                                n2648 = stacked-sequence {
                                tunnel: w4101 -> [_ w4105 _ _]
                                frame #0 {
                                n2649 = property on="Trap Delta (MHz)" class="DigNum (strict)"("Val(Sgnl)"="Move to Delta 2 (MHz)") -> ()  [unwired: 2 in, 2 out]
                                n2650 = case shown="True" "Flow ON after\ntether testing?" {
                                frame False {
                                }
                                frame True {
                                n2651 = property on="Sample Channel\nFlow" class="Bool (strict)"("Val(Sgnl)"=TRUE ("Value (Signaling)")) -> ()  [unwired: 2 in, 2 out]
                                }
                                }
                                }
                                frame #1 {
                                n2652 = flat-sequence {
                                tunnel: w4105 -> [w4107]
                                frame #0 {
                                n2653 = Wait (ms)(milliseconds to wait=u32 500) -> ()  [unwired: 1 out]
                                }
                                frame #1 {
                                n2654 = case shown="\"6\"" w4107 {
                                frame Default {
                                }
                                frame "6" {
                                n2655 = property on="Vortran Laser ON" class="Bool (strict)"("Val(Sgnl)"=TRUE ("Green Laser ON/Interlacing")) -> ()  [unwired: 2 in, 2 out]
                                }
                                }
                                }
                                frame #2 {
                                n2656 = Wait (ms)(milliseconds to wait=u32 500) -> ()  [unwired: 1 out]
                                }
                                frame #3 {
                                n2657 = local write "Start Saving"("Save at end (5, 6)") -> ()
                                }
                                }
                                }
                                frame #2 {
                                n2658 = local read "Bead Sep. Int. Time (s)"() -> (w4113:dbl)
                                n2659 = Multiply(x=w4113, y=1000.0) -> (x*y=w4112:dbl)
                                n2660 = Wait (ms)(milliseconds to wait=w4112) -> ()  [unwired: 1 out]
                                }
                                frame #3 {
                                n2661 = property on="Remove Offset" class="Bool (strict)"("Val(Sgnl)"=TRUE ("Value (Signaling)")) -> ()  [unwired: 2 in, 2 out]
                                }
                                }
                                }
                                }
                                }
                                }
                                }
                                }
                                }
                                frame "2", Default {
                                }
                              }
                            }
                          }
                        }
                      }
                      "Tether" <- "Tether Alarm?"
                    }
                  }
                }
                frame #2 {
                  n2662 = local read "Oscillate Set 1"() -> (w4120:bool)
                  n2663 = local read "Stop All"() -> (w4118:bool)
                  n2664 = Or(x=w4120, y=w4115) -> (x .or. y?=w4117:bool)
                  n2665 = Not(x=w4117) -> (.not. x?=w4119:bool)
                  n2666 = Compound Arithmetic op=OR(w4118, w4119) -> (w4116:bool)
                }
              }
              n2667 = node-c288() -> ()  [unwired: 2 out]
            }
            n2668 = node-c288(w3950) -> ()  [unwired: 1 out]
          }
        }
      }
      event "Fl. Triggered...": Value Change {
        n2669 = event-data() -> ()  [unwired: 7 out]
        n2670 = case shown="True" "Fl. Triggered..." {
          frame False {
          }
          frame True {
            n2671 = node-c288() -> (w4131:T43)  [unwired: 4 out]
            n2672 = timed-loop {
              timing: w4131 -> [_]
              timing-out: [_] -> w4130
              tunnel: "Action" -> [w4139]
              shift-right: [w4136] -> _
              shift-left: u8 255 -> [w4138]
              shift-right: [w4133] -> _
              shift-left: 255 -> [w4135]
              stop <- w4132 stop-if-true
              # "Reset confocal spot"
              n2673 = node-c288() -> ()  [unwired: 2 out]
              n2674 = flat-sequence {
                tunnel: w4139 -> [w4159]
                tunnel: w4138 -> [w4158]
                tunnel: [w4157] -> w4137
                tunnel: w4135 -> [w4144]
                tunnel: [w4143] -> w4134
                tunnel: [w4538] -> w4132
                tunnel: w4137 -> [w4537]
                tunnel: [w4537] -> w4136
                tunnel: [w4536] -> w4133
                tunnel: w4134 -> [w4536]
                frame #0 {
                  n2675 = local read "Delta Fl. 2"() -> (w4156:dbl)
                  n2676 = local read "Delta Fl. 1"() -> (w4151:dbl)
                  n2677 = Multiply(x="Fl. Delta Thresh. (kHz)", y=1000.0) -> (x*y=w4146:dbl)
                  n2678 = Select(t=w4151, s="APD to Watch", f=w4156) -> (s? t:f=w4147:dbl)
                  n2679 = Greater?(x=w4147, y=w4146) -> (0:w4152:bool)
                  n2680 = Or(x="Force Yank", y=w4152) -> (x .or. y?=w4150:bool)
                  n2681 = And(x=w4150, y="Yank when?") -> (x .and. y?=w4148:bool)
                  n2682 = case shown="False" w4148 {
                    tunnel: w4159 -> [w4162 w4363]
                    tunnel: w4158 -> [w4164 w4359]
                    tunnel: [w4164 w4357] -> w4157
                    tunnel: w4147 -> [w4170 _]
                    tunnel: w4146 -> [w4169 _]
                    tunnel: "Force Yank" -> [w4167 _]
                    tunnel: w4144 -> [w4166 w4356]
                    tunnel: [w4165 w4356] -> w4143
                    frame False {
                      n2683 = Negate(x=w4169) -> (-x=w4161:dbl)
                      n2684 = local write "Fl. High"(TRUE ("Fl. High")) -> ()
                      n2685 = Less?(x=w4170, y=w4161) -> (x < y?=w4168:bool)
                      n2686 = Or(x=w4167, y=w4168) -> (x .or. y?=w4163:bool)
                      n2687 = case shown="True" w4163 {
                        tunnel: w4166 -> [w4171 w4181]
                        tunnel: [w4171 w4180] -> w4165
                        tunnel: w4162 -> [_ w4179]
                        frame False {
                        }
                        frame True {
                          n2688 = flat-sequence {
                            tunnel: w4181 -> [w4187]
                            tunnel: w4179 -> [w4184]
                            tunnel: [w4186] -> w4178
                            tunnel: [w4185] -> w4177
                            tunnel: [w4184] -> w4176
                            tunnel: w4175 -> [w4183]
                            tunnel: [w4183] -> w4174
                            tunnel: w4173 -> [w4182]
                            tunnel: [w4182] -> w4172
                            tunnel: [w4258] -> w4180
                            tunnel: w4178 -> [w4258]
                            tunnel: w4177 -> [w4257]
                            tunnel: w4176 -> [w4256]
                            tunnel: w4174 -> [w4255]
                            tunnel: w4172 -> [w4254]
                            frame #0 {
                              n2689 = call <vilib>:"Beep.vi"() -> ()  [unwired: 12 in]
                              n2690 = local write "Waiting"(FALSE ("Waiting")) -> ()
                              n2691 = Increment(x=w4187) -> (x+1=w4186:i32)
                              n2692 = case shown="\"Yank\"" w4184 {
                                tunnel: w4186 -> [_ w4192 _]
                                frame "Alarm", Default {
                                }
                                frame "Yank" {
                                n2693 = flat-sequence {
                                tunnel: w4192 -> [w4195]
                                tunnel: [w4194] -> w4191
                                tunnel: [w4193] -> w4190
                                tunnel: w4191 -> [w4205]
                                tunnel: w4190 -> [w4206]
                                frame #0 {
                                n2694 = local read "Yank Delay (s)"() -> (w4198:dbl)
                                n2695 = local read "N Array El"() -> (w4193:u8)
                                n2696 = Quotient & Remainder(x=w4195, y=w4193) -> (x-y*floor(x/y)=w4194:i32)  [unwired: 1 out]
                                n2697 = Multiply(x=w4198, y=1000.0) -> (x*y=w4196:dbl)
                                n2698 = Wait (ms)(milliseconds to wait=w4196) -> ()  [unwired: 1 out]
                                }
                                frame #1 {
                                n2699 = local read "Yank to which?"() -> (w4200:bool)
                                n2700 = local read "Random Choice"() -> (w4210:bool)
                                n2701 = local read "Yank to Trap Delta (MHz)"() -> (w4203:dbl[])
                                n2702 = local read "Yank to SP"() -> (w4204:dbl[])
                                n2703 = Random Number (0-1)() -> (number: 0 to 1=w4209:dbl)
                                n2704 = Multiply(x=w4206, y=w4209) -> (x*y=w4208:dbl)
                                n2705 = Round Toward -Infinity(1:w4208) -> (0:w4207:dbl)
                                n2706 = Select(t=w4207, s=w4210, f=w4205) -> (s? t:f=w4201:dbl)
                                n2707 = Select(t=w4203, s=w4200, f=w4204) -> (s? t:f=w4202:dbl[])
                                n2708 = Index Array(array=w4202, index=w4201) -> (element=w4199:dbl)
                                n2709 = case shown="False" w4200 {
                                tunnel: w4199 -> [w4211 w4238]
                                frame False {
                                n2710 = flat-sequence {
                                tunnel: w4211 -> [w4212]
                                frame #0 {
                                n2711 = property on="Trap Pos FB SP" class="DigNum (strict)"("Val(Sgnl)"=w4212) -> ()  [unwired: 2 in, 2 out]
                                }
                                frame #1 {
                                n2712 = Wait (ms)(milliseconds to wait=u32 700) -> ()  [unwired: 1 out]
                                }
                                frame #2 {
                                n2713 = local read "Action (%)"() -> (w4217:dbl)
                                n2714 = Absolute Value(x=w4217) -> (abs(x)=w4216:dbl)
                                n2715 = Greater?(x=w4216, y=70.0) -> (0:w4214:bool)
                                n2716 = property on="Remove Action Offset" class="Bool (strict)"("Val(Sgnl)"=w4214) -> ()  [unwired: 2 in, 2 out]
                                }
                                frame #3 {
                                n2717 = for {
                                N: 4 -> [_]
                                n2718 = flat-sequence {
                                frame #0 {
                                n2719 = Wait (ms)(milliseconds to wait=u32 500) -> ()  [unwired: 1 out]
                                }
                                frame #1 {
                                n2720 = local read "Action (%)"() -> (w4223:dbl)
                                n2721 = Absolute Value(x=w4223) -> (abs(x)=w4222:dbl)
                                n2722 = Greater?(x=w4222, y=70.0) -> (0:w4220:bool)
                                n2723 = property on="Remove Action Offset" class="Bool (strict)"("Val(Sgnl)"=w4220) -> ()  [unwired: 2 in, 2 out]
                                }
                                }
                                }
                                }
                                frame #4 {
                                n2724 = Wait (ms)(milliseconds to wait=u32 500) -> ()  [unwired: 1 out]
                                }
                                frame #5 {
                                n2725 = local read "Mean"() -> (w4231:dbl)
                                n2726 = Greater?(x=w4231, y=11.0) -> (0:w4225:bool)
                                n2727 = Not(x=w4225) -> (.not. x?=w4226:bool)
                                n2728 = And(x=w4226, y="Shift confocal") -> (x .and. y?=w4228:bool)
                                n2729 = And(x=w4225, y="Shift confocal") -> (x .and. y?=w4229:bool)
                                n2730 = case shown="True" w4229 {
                                frame False {
                                }
                                frame True {
                                n2731 = local read "Confocal Y 2 (V)"() -> (w4235:dbl)
                                n2732 = local read "Confocal X 2 (V)"() -> (w4234:dbl)
                                n2733 = property on="AO1" class="Slide (strict)"("Val(Sgnl)"=w4235) -> ()  [unwired: 2 in, 2 out]
                                n2734 = property on="AO2" class="Slide (strict)"("Val(Sgnl)"=w4234) -> ()  [unwired: 2 in, 2 out]
                                }
                                }
                                n2735 = case shown="True" w4228 {
                                frame False {
                                }
                                frame True {
                                n2736 = local read "Confocal Y 1 (V)"() -> (w4233:dbl)
                                n2737 = local read "Confocal X 1 (V)"() -> (w4232:dbl)
                                n2738 = property on="AO1" class="Slide (strict)"("Val(Sgnl)"=w4233) -> ()  [unwired: 2 in, 2 out]
                                n2739 = property on="AO2" class="Slide (strict)"("Val(Sgnl)"=w4232) -> ()  [unwired: 2 in, 2 out]
                                }
                                }
                                }
                                frame #6 {
                                n2740 = Wait (ms)(milliseconds to wait=u32 1500) -> ()  [unwired: 1 out]
                                }
                                frame #7 {
                                n2741 = property on="Rem fb disp offset" class="Bool (strict)"("Val(Sgnl)"=TRUE ("Value (Signaling)")) -> ()  [unwired: 2 in, 2 out]
                                }
                                }
                                }
                                frame True {
                                n2742 = flat-sequence {
                                tunnel: w4238 -> [w4239]
                                frame #0 {
                                n2743 = property on="Trap Delta (MHz)" class="DigNum (strict)"("Val(Sgnl)"=w4239) -> ()  [unwired: 2 in, 2 out]
                                }